vi "Main.vi"() -> ()   [LabVIEW 2020]
uses:
  System.Windows.Forms
  Global_Variable/Global.vi
  Global_Variable/A180648.vi
  <userlib>/_MGI/Menu Building/MenuTypes/MenuStrip/MGI_MenuStrip.lvclass
  <userlib>/_MGI/Menu Building/MenuItemStatusChange/MGI_MenuItemStatusChange.lvclass
  Libraries/S7/S7.lvlib
panel:
  out "上序状态":string
  out "客户软件版本号":string
  in  "Andon":enum32{"未选择", "缺料报警", "质量报警", "故障报警"}(radio)
  out "PLC":bool
  in  "菜单":refnum<k24>(container)
  in  "Result":string[][](table)
  out "逆向空载":bool
  out "试验计时":u16
  out "产品编号":string
  out "生产数量":i32
  out "合格数量":i32
  out "userStatus":string caption="用户状态"
  out "userName":string caption="用户名"
  out "connectionMode":string caption="联机类型"
  out "产品型号":string
  out "功能":bool
  out "空载":bool
  out "振动NVH":bool
  out "磨合":bool
  out "备用试验2":bool
  out "传感器特性":bool
  out "电流特性":bool
  out "力特性":bool
  in  "更换产品":refnum<vi>
  out "提示信息":string
  out "错误":bool
  out "时间字符串":string
  out "日期字符串":string
  out "自动":bool
  # "NVH噪声检测"
  # "试验项目"
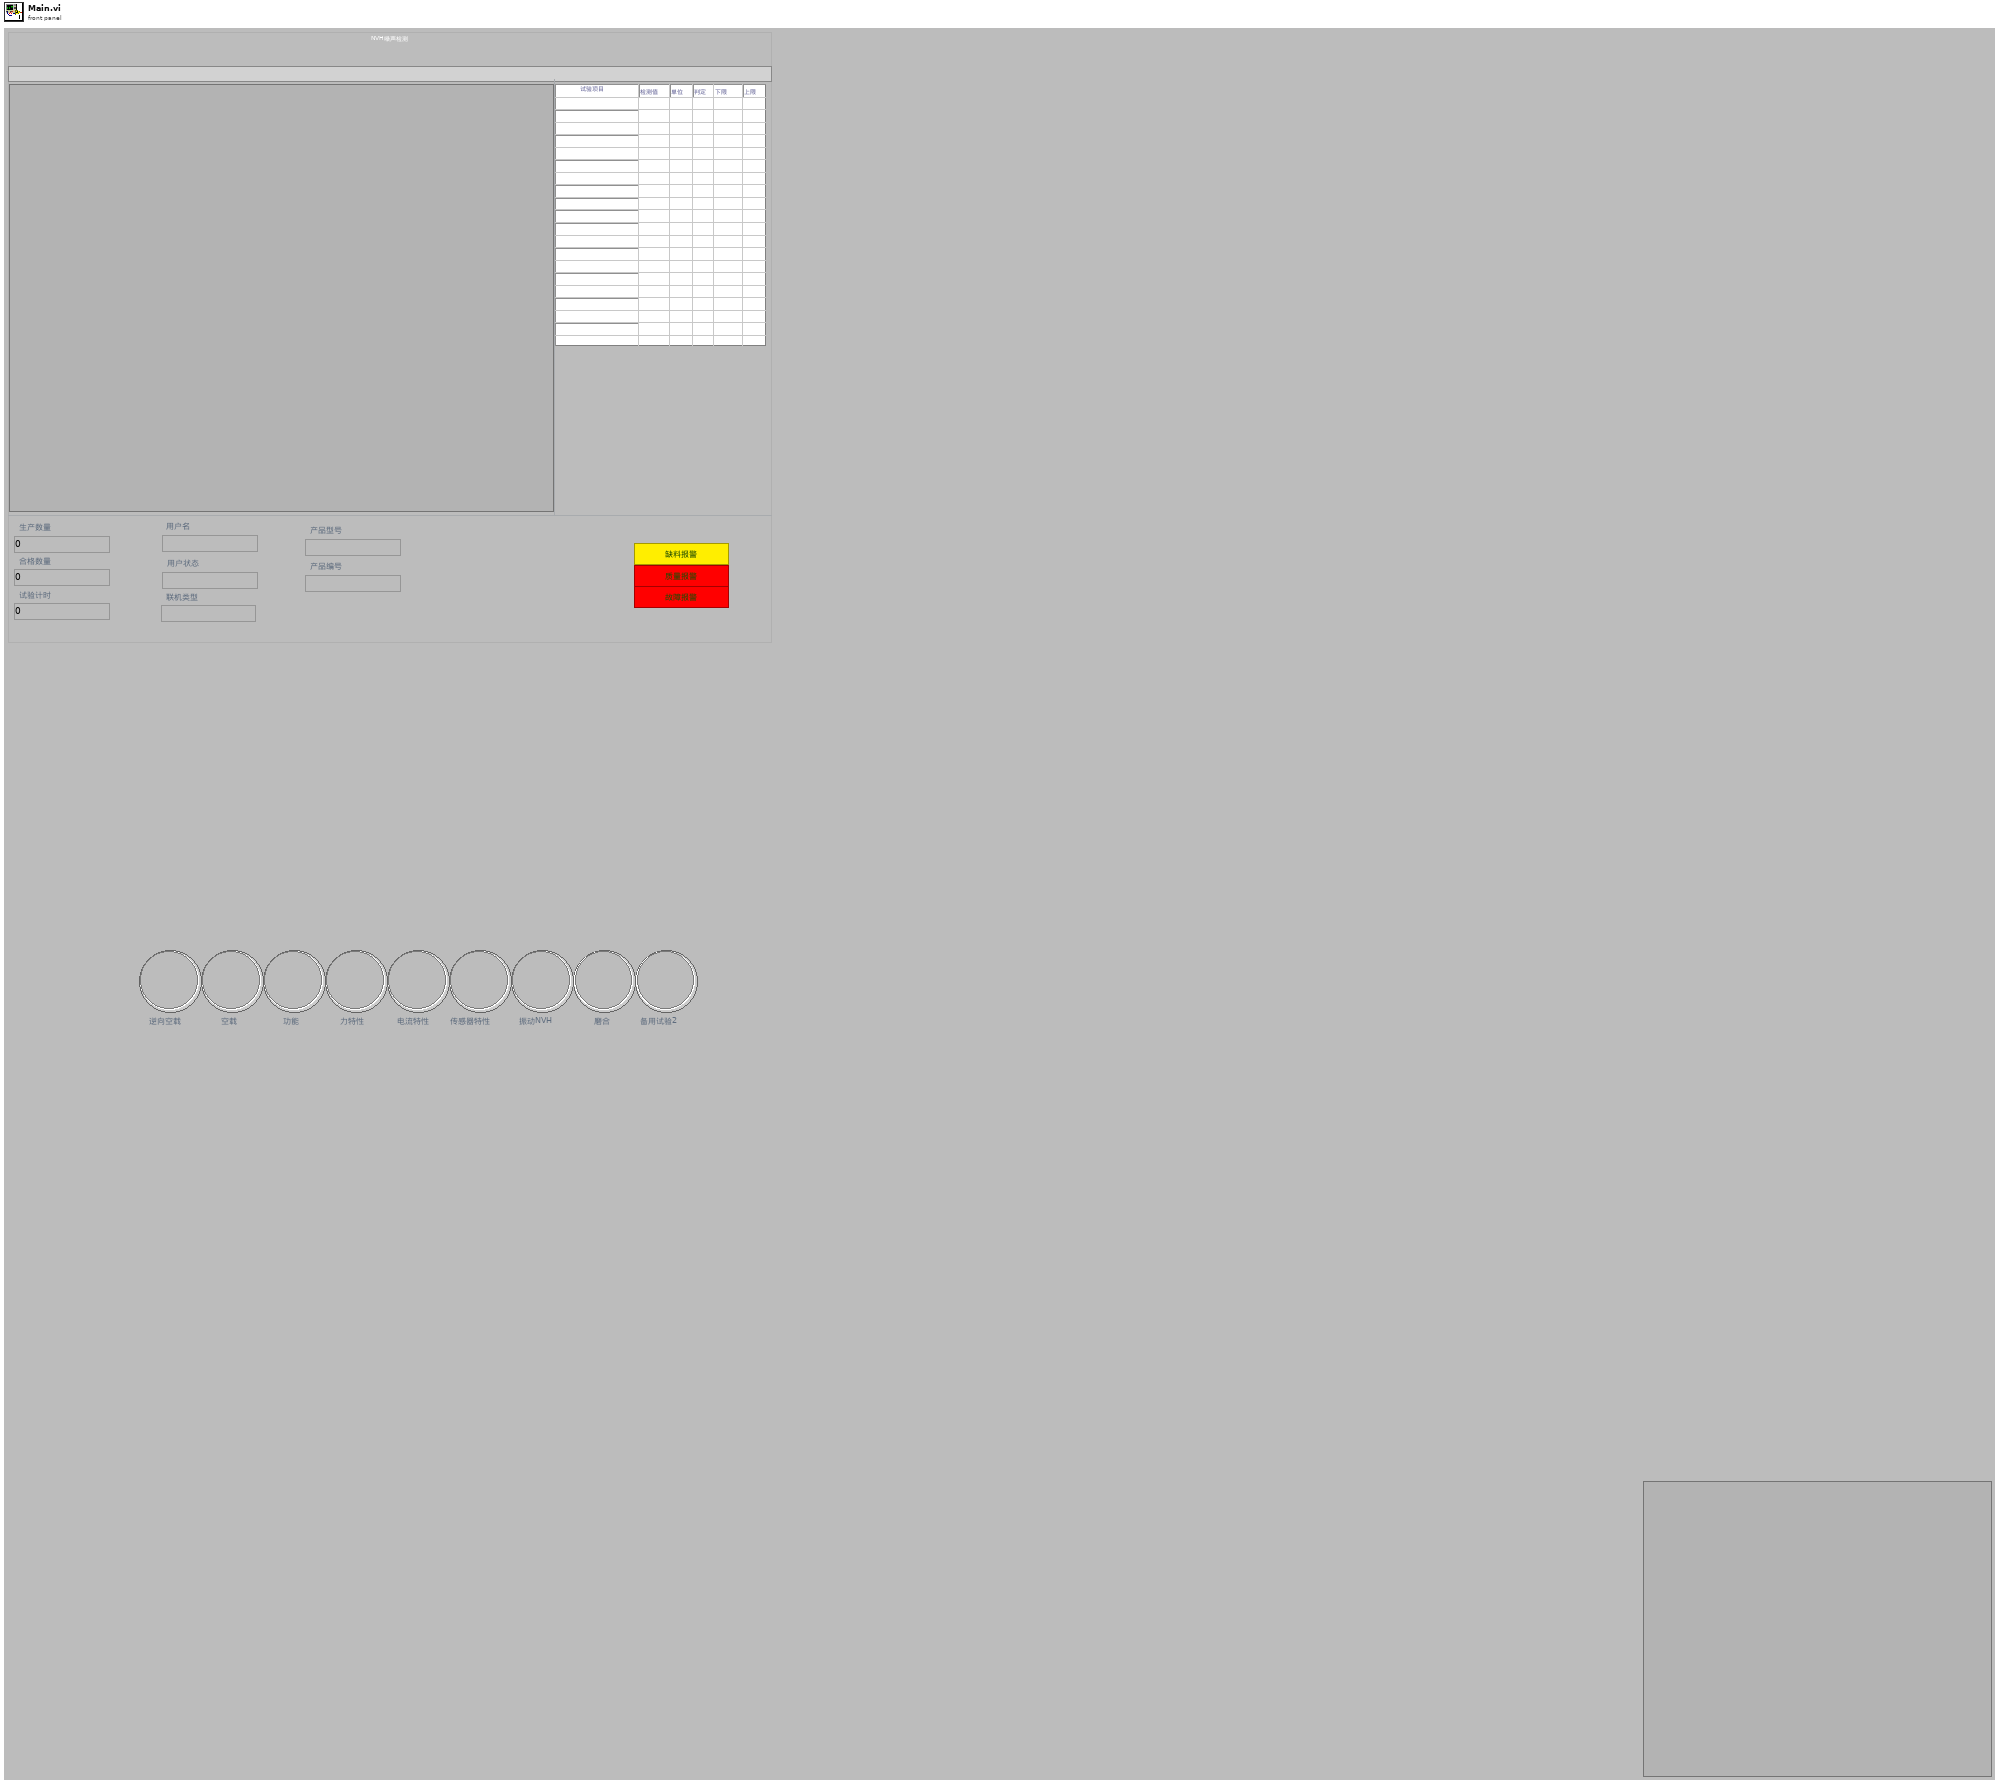
[diagram p1: front panel]
types:
  T1 = typedef "S7.lvlib/Broadcast Events--cluster.ctl" = cluster{"Module Did Init":refnum<user-event>, "Status Updated":refnum<user-event>, "Error Reported":refnum<user-event>, "Module Did Stop":refnum<user-event>, "Update Module Execution Status":refnum<user-event>}
  T2 = enum32{"空载", "功能", "力特性", "电流特性", "传感器特性", "逆向空载", "磨合", "振动NVH"}
  T3 = enum32{"Invalid", "Standard", "Closed", "Hidden", "Minimized", "Maximized"}
  T4 = cluster{"设备名称":string, "操作人员":string, "设备状态":enum16{"设备离线", "设备正常", "设备缺料", "设备故障", "质量报警"}, "附加信息":string}
  T5 = enum32{"invalid app kind", "Development System", "Run Time System", "Student Edition", "Embedded LabVIEW", "Evaluation", "Custom"}
  T6 = cluster{"操作员编号":string, "操作员姓名":string, "操作员权限":string, "联机模式":enum16{"单机", "追溯"}}
  T7 = cluster{"Core":cluster{"Current VI Reference":refnum<vi>, "Close Panel on Exit?":bool}, "Your Boolean data":bool, "Your string data":string}
  T8 = cluster{"Current VI Reference":refnum<vi>, "Close Panel on Exit?":bool}
  T9 = cluster{"用户编号":string, "用户名":string, "用户密码(密文)":string, "用户权限":string}
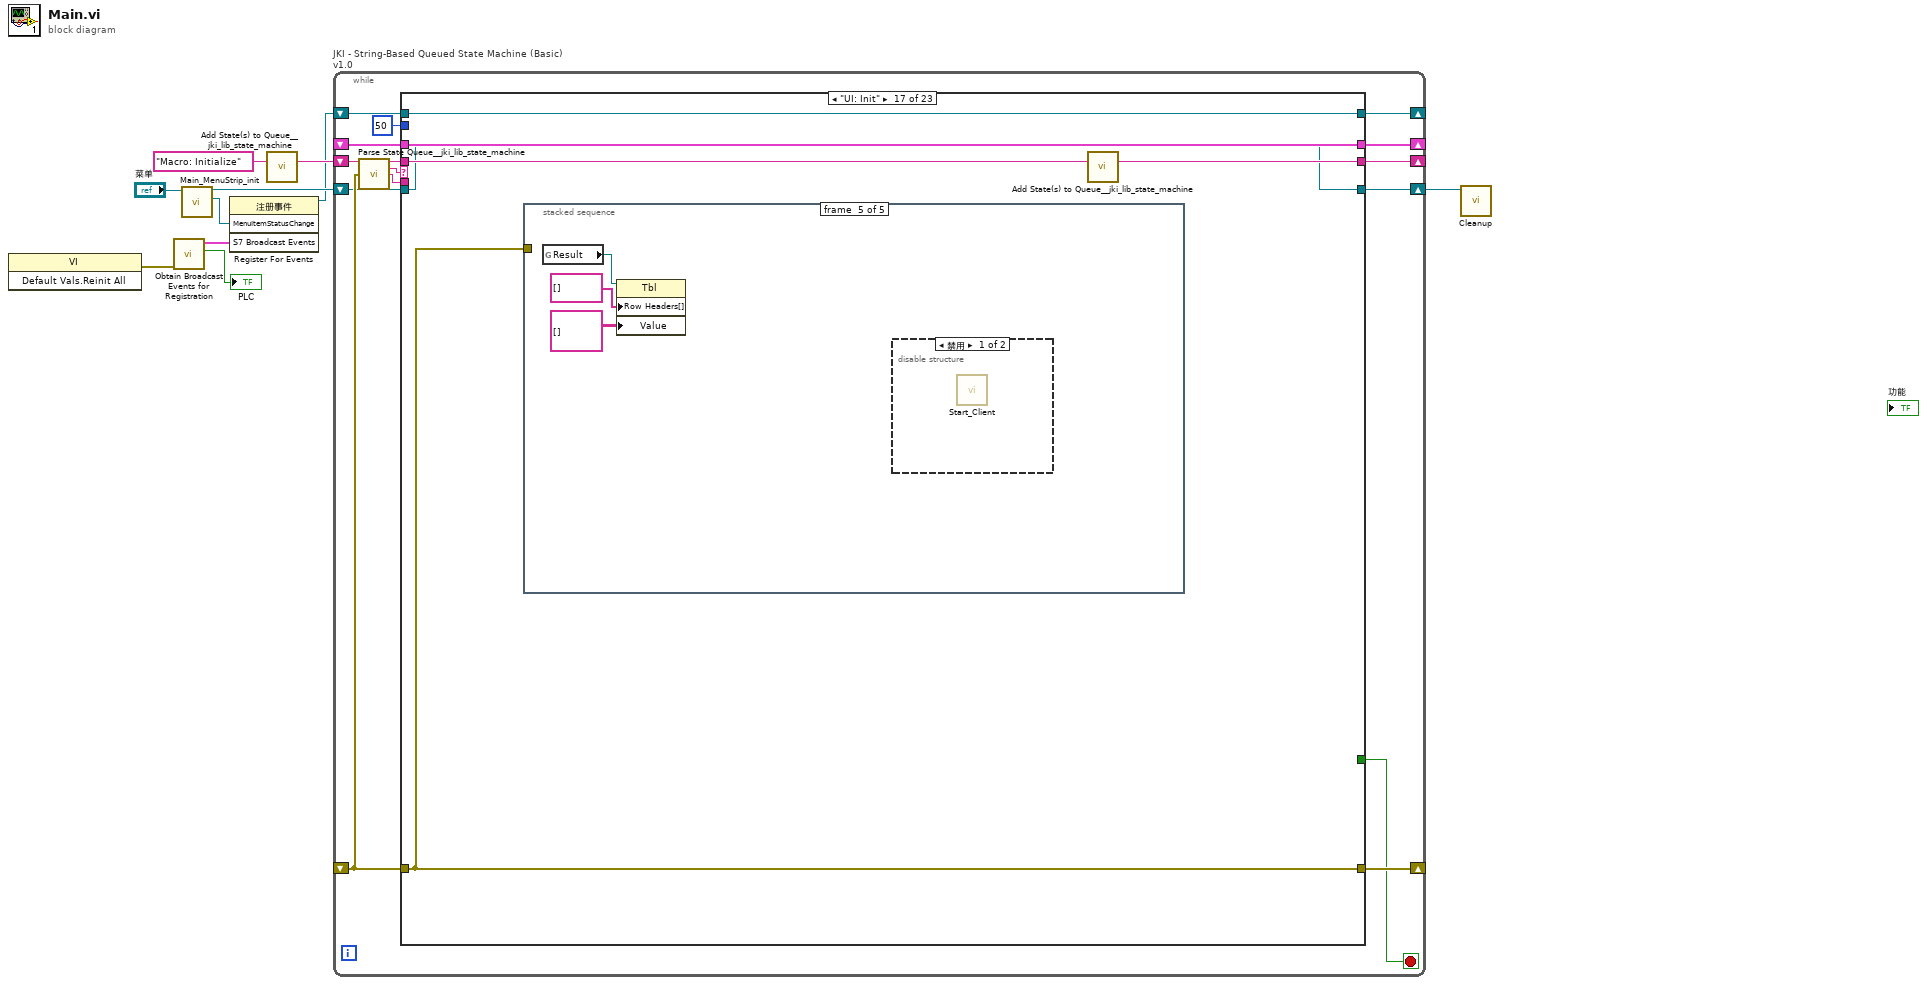
[diagram p0: block diagram]
diagram:
  n1 = invoke class="VI" method="Default Vals.Reinit All"() -> (error out=w3:errorcluster)  [unwired: 3 in, 2 out]
  n2 = call "Obtain Broadcast Events for Registration.vi"("error in (no error)"=w3) -> ("Already running?"=→"PLC":bool, "S7 Broadcast Events"=w5:T1)  [unwired: 8 in, 1 out]
  n3 = call "Main_MenuStrip_init.vi"("MenuStrip"="菜单") -> ("MenuItemStatusChange"=w2:refnum<user-event>, "Menu out"=w7:refnum<class "MGI_MenuStrip.lvclass">)  [unwired: 9 in]
  n4 = register-events(w2, w5) -> (reference out=w1:refnum<event-registration>)  [unwired: 2 in, 1 out]
  n5 = call <vilib>:"Add State(s) to Queue__jki_lib_state_machine.vi"("State(s) in (\"\")"="Macro: Initialize") -> ("States Out"=w10:string)  [unwired: 14 in]
  n6 = while "JKI - String-Based Queued State Machine (Basic) v1.0" {
    shift-right: [w19] -> _
    shift-left: _ -> [w18]
    shift-right: [w21] -> _
    shift-left: _ -> [w16]
    shift-right: [w20] -> _
    shift-left: w10 -> [w22]
    shift-right: [w14] -> w6
    shift-left: w7 -> [w15]
    shift-right: [w12] -> _
    shift-left: w1 -> [w11]
    stop <- w13 stop-if-true
    n7 = call <vilib>:"Parse State Queue__jki_lib_state_machine.vi"("State Queue"=w22, "Error In (no error)"=w16) -> ("Remaining States"=w24:string, "Current State"=w25:string, "Arguments"=w23:string)  [unwired: 11 in]
    n8 = case shown="\"UI: Init\"" w25 {
      selector: w25 -> [_ _ w278 _ _ _ _ _ _ _ _ _ _ _ _ _ _ _ _ _ _ _ _]
      tunnel: w24 -> [w36 w275 w282 w302 w310 w318 w324 w328 w334 w340 w346 w355 w366 w374 w380 w387 w411 w448 w456 w469 w497 w504 w517]
      tunnel: w23 -> [_ _ _ _ _ _ _ _ _ _ _ _ _ _ _ _ _ _ w451 w463 _ _ _]
      tunnel: w18 -> [w34 w272 w280 w293 w307 w316 w321 w329 w337 w343 w349 w352 _ w369 w377 w385 w409 w445 w454 w465 w494 w501 w514]
      tunnel: [w33 w273 w284 w299 errorcluster {"status"=FALSE, "code"=0, "source"=""} ("error out") w315 w322 w326 w332 w339 w345 w353 w363 w370 w378 w384 w407 w446 w452 w466 w495 w502 w515] -> w21
      tunnel: w16 -> [w32 w273 w283 w299 w306 w315 w322 w326 w333 w339 w345 w353 w363 w371 w378 w381 w407 w446 w453 w467 w495 w502 w515]
      tunnel: [w35 w274 w281 w301 w309 w317 w323 w328 w335 w341 w347 w354 w365 w373 w379 w386 w410 w447 w455 w468 w496 w503 w516] -> w20
      tunnel: [w31 w272 w280 w300 w307 w316 w321 w329 w337 w343 w349 w352 w364 w369 w377 w385 w409 w445 w454 w465 w494 w501 w514] -> w19
      tunnel: 50 ("Timeout") -> [w30 _ _ _ _ _ _ _ _ _ _ _ _ _ _ _ _ _ _ _ _ _ _]
      tunnel: w15 -> [w29 w271 w277 w290 w304 w314 w320 w327 w336 w342 w348 w351 w357 w368 w376 w383 w408 w444 w450 w462 w493 w499 w507]
      tunnel: [w28 w271 w277 w290 w304 w314 w320 w327 w336 w342 w348 w351 w357 w368 w376 w383 w408 w444 w450 w462 w493 w499 w507] -> w14
      tunnel: [_ _ _ _ _ TRUE _ _ _ _ _ _ _ _ _ _ _ _ _ _ _ _ _] -> w13
      tunnel: [w26 w270 w276 w289 w303 w312 w319 w330 w331 w338 w344 w350 w358 w367 w375 w382 w406 w441 w449 w461 w492 w498 w506] -> w12
      tunnel: w11 -> [w27 w270 w276 w289 w303 w312 w319 w330 w331 w338 w344 w350 w358 w367 w375 w382 w406 w441 w449 w461 w492 w498 w506]
      frame "", "Event Structure", "Idle" {
        n9 = event shown="[8] \"自动\": 鼠标按下" {
          selector: w27 -> [w40 w65 w82 w93 w155 w162 w169 w176 w191 w192 w199 w208 _]
          dyn-events: [w40 w65 w81 w93 w155 w162 w169 w176 w191 w192 w199 w208 _] -> w26
          timeout: w30 -> [_ _ _ _ _ _ _ _ _ _ _ _ _]
          tunnel: w36 -> [w52 w68 w91 w102 w156 w163 w172 w179 w188 w196 w206 w210 w260]
          tunnel: [w51 w67 w91 w100 w157 w164 w173 w180 w189 w197 w205 w211 w260] -> w35
          tunnel: w34 -> [w50 w69 w92 w101 w159 w167 w174 w181 w190 w198 w203 w213 w261]
          tunnel: [w41 w66 w83 w103 w160 w165 w170 w182 w186 w195 w204 w212 w258] -> w33
          tunnel: w32 -> [w41 w66 w84 w103 w160 w165 w170 w183 w186 w195 w204 w212 w258]
          tunnel: [w50 w69 w92 w101 w159 w167 w174 w181 w190 w198 w203 w213 w261] -> w31
          tunnel: w29 -> [w39 _ w90 w96 w158 w166 w171 w178 w187 _ _ _ w259]
          tunnel: [w39 _ w90 w96 w158 w166 w171 w178 w187 _ _ _ w259] -> w28
          event Timeout {
            n10 = event-data() -> ()  [unwired: 1 in, 1 out]
            n11 = global read "Global.vi" "计时开始"() -> (w43:bool)
            n12 = global read "Global.vi" "软件版本号"() -> (→"客户软件版本号":string)
            n13 = case shown="真" w43 {
              frame False {
                n14 = global write "Global.vi" "计时复位"(TRUE ("计时复位")) -> ()
              }
              frame True {
                n15 = stacked-sequence {
                  frame #0 {
                    n16 = global read "Global.vi" "计时复位"() -> (w54:bool)
                    n17 = call "已用时间"("Reset"=w54) -> ("Elapsed Time (s)"=→"试验计时":dbl)  [unwired: 11 in, 7 out]
                  }
                  frame #1 {
                    n18 = global write "Global.vi" "计时复位"(FALSE ("计时复位")) -> ()
                  }
                }
              }
            }
            n19 = Format Date/Time String(time format string (%c)="%H:%M ") -> (date/time string=→"时间字符串":string)  [unwired: 2 in]
            n20 = Format Date/Time String(time format string (%c)="%Y年%m月%d日") -> (date/time string=→"日期字符串":string)  [unwired: 2 in]
            n21 = control-ref of="上序状态"() -> (w37:refnum<vi>)
            n22 = call <vilib>:"Add State(s) to Queue__jki_lib_state_machine.vi"("State(s) in (\"\")"=w52) -> ("States Out"=w51:string)  [unwired: 14 in]
            n23 = global read "Global.vi" "合格数量"() -> (→"合格数量":i32)
            n24 = global write "Global.vi" "提示信息"(w37) -> ()
            n25 = global read "Global.vi" "生产数量"() -> (→"生产数量":i32)
            n26 = global read "Global.vi" "产品编号"() -> (→"产品编号":string)
          }
          event "空载", "功能", "力特性", "传感器特性", "电流特性", "振动NVH", "逆向空载", "磨合": Mouse Down {
            w57 = refnum<user-event> refnum items=["空载", "功能", "力特性", "电流特性", "传感器特性", "逆向空载", "磨合", "振动NVH"] ("试验项_Event")
            n27 = event-data() -> ("CtlRef"=w60:refnum<vi>)  [unwired: 1 in]
            n28 = property class="Bool (严格)"(reference=w60) -> ("Label.Text"=w59:string)  [unwired: 1 in, 2 out]
            n29 = vi-ref "Auto.vi"() -> (w63:refnum<vi>)
            n30 = case shown="\"磨合\"" w59 {
              tunnel: [T2."空载" ("事件数据") T2."功能" ("事件数据") T2."力特性" ("事件数据") T2."传感器特性" ("事件数据") T2."电流特性" ("事件数据") T2."逆向空载" ("事件数据") T2."磨合" ("事件数据") T2."振动NVH" ("事件数据")] -> w58
              frame "空载", Default {
              }
              frame "功能" {
              }
              frame "力特性" {
              }
              frame "传感器特性" {
              }
              frame "电流特性" {
              }
              frame "逆向空载" {
              }
              frame "磨合" {
              }
              frame "振动NVH" {
              }
            }
            n31 = invoke class="VI" method="Ctrl Val.Get"(reference=w63, "Control Name"="试验项_Event" ("控件名")) -> ("Get Control Value Variant"=w62:variant)  [unwired: 2 in, 3 out]
            n32 = Variant To Data(type=w57, Variant=w62) -> (data=w61:refnum<user-event>)  [unwired: 1 in, 1 out]
            n33 = Generate User Event(user event=w61, event data cluster=w58) -> ()  [unwired: 2 in, 2 out]
            n34 = call <vilib>:"Add State(s) to Queue__jki_lib_state_machine.vi"("State(s) in (\"\")"=w68) -> ("States Out"=w67:string)  [unwired: 14 in]
          }
          event "PLC": Value Change; "PLC": Mouse Down {
            n35 = event-data() -> ()  [unwired: 1 in, 4 out]
            n36 = call "Start Module.vi"("error in (no error)"=w84) -> ("error out"=w80:errorcluster, "Wait for Event Sync?"=w89:bool, "S7 Broadcast Events"=w88:T1, "Module Was Already Running?"=w87:bool)  [unwired: 7 in]
            n37 = local write "PLC"(w87) -> ()
            n38 = register-events(reference=w82, error in=w80, w88) -> (reference out=w81:refnum<event-registration>, error out=w79:errorcluster)  [unwired: 1 in]
            n39 = call "Synchronize Module Events.vi"("error in (no error)"=w79, "Wait for Event Sync?"=w89) -> ("error out"=w78:errorcluster)  [unwired: 9 in]
            n40 = call "Init S7 Link.vi"("error in (no error)"=w78, "超时"=500, "IP"="192.168.0.61") -> ("error out"=w83:errorcluster)  [unwired: 8 in]
          }
          event User Event {
            n41 = event-data() -> ("StatusChange"=w94:refnum<class "MGI_MenuItemStatusChange.lvclass">)  [unwired: 1 in]
            n42 = call <userlib>:"BasicInfo.vi"("MGI_MenuItemStatusChange in"=w94) -> ("Enabled?"=w97:bool, "Checked?"=w98:bool, "Tag"=w99:string)  [unwired: 7 in, 1 out]
            n43 = case shown="\"关于\"" w99 {
              tunnel: w98 -> [_ _ _ _ _ _ _ _ _ _ _ _ _ _ _]
              tunnel: w97 -> [_ _ _ _ _ _ _ _ _ _ _ _ _ _ _]
              tunnel: [_ _ "S7: Stop\nCAN: Stop\nMacro: Exit" _ _ _ _ _ _ _ _ _ _ _ _] -> w95
              frame "假", Default {
              }
              frame "数据库配置" {
                n44 = global read "用户信息.vi" "用户信息"() -> (w105:T6)
                n45 = Unbundle By Name(w105) -> ("操作员权限"=w104:string)
                n46 = case shown="\"系统管理员\"" w104 {
                  frame Default {
                    n47 = One Button Dialog(message="权限不足！" ("消息")) -> ()  [unwired: 1 in, 1 out]
                  }
                  frame "系统管理员" {
                    n48 = vi-ref "数据库配置.vi"() -> (w108:refnum<vi>)
                    n49 = call "CallVI.vi"("VI引用"=w108, "状态"=T3."Standard") -> ()  [unwired: 12 in, 2 out]
                  }
                }
              }
              frame "退出" {
                n50 = global write "Global.vi" "程序关闭"(TRUE ("程序关闭")) -> ()
                n51 = call "Close_Client.vi"() -> ()  [unwired: 12 in]
              }
              frame "手动控制" {
                n52 = global read "用户信息.vi" "用户信息"() -> (w112:T6)
                n53 = Unbundle By Name(w112) -> ("操作员权限"=w111:string)
                n54 = case shown="\"班组长\", \"系统管理员\"" w111 {
                  frame Default {
                    n55 = One Button Dialog(message="权限不足！" ("消息")) -> ()  [unwired: 1 in, 1 out]
                  }
                  frame "班组长", "系统管理员" {
                  }
                }
              }
              frame "半自动控制" {
                n56 = disable-structure shown="启用" {
                  frame Disabled {
                    n57 = shared-variable "我的电脑\\Global.lvlib\\操作者权限"() -> (w114:string)  [unwired: 1 in, 1 out]
                    n58 = case shown="\"班组长\", \"系统管理员\"" w114 {
                      frame Default {
                        n59 = One Button Dialog(message="权限不足！" ("消息")) -> ()  [unwired: 1 in, 1 out]
                      }
                      frame "班组长", "系统管理员" {
                        n60 = call "CallVI.vi"("VI引用"=refnum<vi> refnum, "状态"=T3."Maximized") -> ()  [unwired: 12 in, 2 out]
                      }
                    }
                  }
                  frame Enabled {
                    n61 = One Button Dialog(message="当前设备不具备半自动功能！" ("消息")) -> ()  [unwired: 1 in, 1 out]
                  }
                }
              }
              frame "产品管理" {
                n62 = vi-ref "Config.vi"() -> (w120:refnum<vi>)
                n63 = call "CallVI.vi"("VI引用"=w120, "状态"=T3."Standard") -> ()  [unwired: 12 in, 2 out]
              }
              frame "系统配置" {
                n64 = global read "用户信息.vi" "用户信息"() -> (w122:T6)
                n65 = Unbundle By Name(w122) -> ("操作员权限"=w121:string)
                n66 = case shown="\"班组长\", \"系统管理员\"" w121 {
                  frame Default {
                    n67 = One Button Dialog(message="权限不足！" ("消息")) -> ()  [unwired: 1 in, 1 out]
                  }
                  frame "班组长", "系统管理员" {
                  }
                }
              }
              frame "用户管理" {
                n68 = global read "用户信息.vi" "用户信息"() -> (w125:T6)
                n69 = Unbundle By Name(w125) -> ("操作员权限"=w124:string)
                n70 = case shown="\"系统管理员\"" w124 {
                  frame Default {
                    n71 = One Button Dialog(message="权限不足！" ("消息")) -> ()  [unwired: 1 in, 1 out]
                  }
                  frame "系统管理员" {
                    n72 = vi-ref "User_manager.vi"() -> (w128:refnum<vi>)
                    n73 = call "CallVI.vi"("VI引用"=w128, "状态"=T3."Standard") -> ()  [unwired: 12 in, 2 out]
                  }
                }
              }
              frame "编码规则" {
                n74 = global read "用户信息.vi" "用户信息"() -> (w130:T6)
                n75 = Unbundle By Name(w130) -> ("操作员权限"=w129:string)
                n76 = case shown="\"班组长\", \"工艺管理员\", \"系统管理员\"" w129 {
                  frame Default {
                    n77 = One Button Dialog(message="权限不足！" ("消息")) -> ()  [unwired: 1 in, 1 out]
                  }
                  frame "班组长", "工艺管理员", "系统管理员" {
                    n78 = vi-ref "编码规则设置.vi"() -> (w133:refnum<vi>)
                    n79 = call "CallVI.vi"("VI引用"=w133, "状态"=T3."Standard") -> ()  [unwired: 12 in, 2 out]
                  }
                }
              }
              frame "易损件管理" {
                n80 = vi-ref "易损件管理.vi"() -> (w135:refnum<vi>)
                n81 = call "CallVI.vi"("VI引用"=w135, "状态"=T3."Standard") -> ()  [unwired: 12 in, 2 out]
              }
              frame "物料批次管理" {
                n82 = vi-ref "批次管理.vi"() -> (w137:refnum<vi>)
                n83 = call "CallVI.vi"("VI引用"=w137, "状态"=T3."Standard") -> ()  [unwired: 12 in, 2 out]
              }
              frame "报表" {
                n84 = call "文件对话框"("start path"=path "D:/report", "prompt"="打开报表", "pattern (all files)"="*.doc;*.docx", "pattern label"="Word 文档") -> ("selected path"=w138:path, "error out"=w139:errorcluster)  [unwired: 8 in, 2 out]
                n85 = case shown="无错误" w139 {
                  selector: w139 -> [w145 w147]
                  tunnel: w138 -> [w146 _]
                  frame No Error {
                    w144 = 1 items=["Normal", "Maximize", "Minimize"] ("cpubbs_WindowState")
                    n86 = call "Open_Word.vi"("File Path"=w146, "cpubbs_WindowState"=w144, "错误输入（无错误）"=w145) -> ()  [unwired: 12 in, 1 out]
                  }
                  frame Error {
                    n87 = call <vilib>:"Clear Errors.vi"("error in (no error)"=w147) -> ()  [unwired: 5 in, 2 out]
                  }
                }
              }
              frame "报警信息" {
                n88 = vi-ref "报警信息.vi"() -> (w149:refnum<vi>)
                n89 = call "CallVI.vi"("VI引用"=w149, "状态"=T3."Standard") -> ()  [unwired: 12 in, 2 out]
              }
              frame "关于" {
                n90 = vi-ref "About.vi"() -> (w151:refnum<vi>)
                n91 = call "CallVI.vi"("VI引用"=w151, "状态"=T3."Standard") -> ()  [unwired: 12 in, 2 out]
              }
              frame "操作演示" {
                n92 = call <vilib>:"Application Directory.vi"() -> ("Application Directory"=w154:path)
                n93 = Build Path(base path=w154, name or relative path="操作演示" ("名称或相对路径")) -> (appended path=w153:path)
                n94 = call "自动播放ppt.vi"("路径"=w153) -> ()  [unwired: 10 in, 1 out]
              }
            }
            n95 = call <vilib>:"Add State(s) to Queue__jki_lib_state_machine.vi"("State(s) in (\"\")"=w102, "State(s) at Back (\"\")"=w95) -> ("States Out"=w100:string)  [unwired: 13 in]
          }
          event User Event {
            n96 = event-data() -> ("Init?"=w161:bool)  [unwired: 1 in, 1 out]
            n97 = local write "PLC"(w161) -> ()
            n98 = call <vilib>:"Add State(s) to Queue__jki_lib_state_machine.vi"("State(s) in (\"\")"=w156) -> ("States Out"=w157:string)  [unwired: 14 in]
          }
          event User Event {
            n99 = event-data() -> ("Running?"=w168:bool)  [unwired: 1 in]
            n100 = local write "PLC"(w168) -> ()
            n101 = call <vilib>:"Add State(s) to Queue__jki_lib_state_machine.vi"("State(s) in (\"\")"=w163) -> ("States Out"=w164:string)  [unwired: 14 in]
          }
          event User Event {
            n102 = event-data() -> ()  [unwired: 1 in, 7 out]
            n103 = local write "PLC"(FALSE ("PLC")) -> ()
            n104 = call <vilib>:"Add State(s) to Queue__jki_lib_state_machine.vi"("State(s) in (\"\")"=w172) -> ("States Out"=w173:string)  [unwired: 14 in]
          }
          event User Event {
            n105 = event-data() -> ("Error"=w184:errorcluster)  [unwired: 1 in]
            n106 = Merge Errors(w184, w183) -> (w182:errorcluster)
            n107 = disable-structure shown="禁用" {
              disable-tunnel: ["S7: Stop\nS7: Initialize\nIdle" _] -> w177
              frame Disabled {
              }
              frame Enabled {
              }
            }
            n108 = call <vilib>:"Add State(s) to Queue__jki_lib_state_machine.vi"("State(s) in Front (\"\")"=w177, "State(s) in (\"\")"=w179) -> ("States Out"=w180:string)  [unwired: 13 in]
          }
          event "自动": Mouse Down {
            n109 = event-data() -> ()  [unwired: 1 in, 1 out]
            n110 = call <vilib>:"Add State(s) to Queue__jki_lib_state_machine.vi"("State(s) in (\"\")"=w188) -> ("States Out"=w189:string)  [unwired: 14 in]
          }
          event "错误": Mouse Down {
            n111 = event-data() -> ()  [unwired: 1 in, 8 out]
            n112 = vi-ref "报警信息.vi"() -> (w194:refnum<vi>)
            n113 = call "CallVI.vi"("VI引用"=w194, "状态"=T3."Standard") -> ()  [unwired: 12 in, 2 out]
            n114 = call <vilib>:"Add State(s) to Queue__jki_lib_state_machine.vi"("State(s) in (\"\")"=w196) -> ("States Out"=w197:string)  [unwired: 14 in]
          }
          event Panel Close? {
            n115 = event-data() -> ()  [unwired: 1 in, 1 out]
            n116 = disable-structure shown="禁用" {
              frame Disabled {
                n117 = call "Close.vi"() -> ()  [unwired: 11 in, 1 out]
              }
              frame Enabled {
              }
            }
            n118 = global write "Global.vi" "程序关闭"(TRUE ("程序关闭")) -> ()
            n119 = call <vilib>:"Add State(s) to Queue__jki_lib_state_machine.vi"("State(s) in Front (\"\")"="S7: Stop\nMacro: Exit", "State(s) in (\"\")"=w206) -> ("States Out"=w205:string)  [unwired: 13 in]
            n120 = event-data("Discard?"=TRUE) -> ()  [unwired: 1 in, 1 out]
          }
          event "更换产品": Value Change {
            n121 = event-data() -> ("NewVal"=w209:refnum<vi>)  [unwired: 1 in, 5 out]
            n122 = stacked-sequence {
              tunnel: w209 -> [w215]
              tunnel: [w214] -> w207
              frame #0 {
                n123 = stacked-sequence {
                  tunnel: w215 -> [w223 _ _]
                  tunnel: [_ w227 _] -> w214
                  frame #0 {